vi "UHR-Fleezers Control (host) - 12.7c.vi"() -> ()   [LabVIEW 2012] (continued)
      tunnel: [w1052 _ _ _ w1081 _ w1113 _ _ w1145 _ w1159 _ _ w1229 w1232 w1242 w1245 w1315 _ w1336 w1361 w1381 w1402 w1422 w1447 w1477 _ w1484 w1579 w1584 w1622 _ w1657 w1661 w1665 w1676 w1680 _ w1688 _ _ _ _ _ _ _ _ _ _ _ _ _ _ _ _ _ w2066 _ _ _ _ w2107 _ _ _ _ _ _ _ _ _ _ _] -> w1011
      tunnel: w1010 -> [w1051 _ _ _ w1090 _ w1112 _ _ w1145 _ w1179 _ _ w1228 w1231 w1241 w1244 w1320 _ w1335 w1360 w1382 w1403 w1423 w1452 w1478 w1481 w1485 w1580 w1585 w1623 _ w1658 w1662 w1673 w1677 w1681 _ w1689 _ _ _ _ _ _ _ _ _ _ _ _ _ _ _ _ _ w2067 _ w2084 _ w2091 w2109 _ w2116 w2124 w2139 w2155 w2161 _ w2170 _ w2189 _]
      tunnel: [_ _ _ _ _ _ _ _ _ w1144 _ _ _ _ _ _ _ _ _ _ _ _ _ _ _ _ _ _ _ _ _ _ _ _ _ _ _ _ _ _ _ _ _ _ _ _ _ _ _ _ _ _ _ _ _ _ _ _ _ _ _ _ _ _ _ _ _ _ _ _ _ _ _ _] -> w1009
      tunnel: [_ _ _ _ _ _ _ "Round T1 X" _ _ _ _ _ _ _ _ _ _ _ _ _ _ _ _ _ _ _ _ _ _ _ _ _ _ _ _ _ _ _ _ _ _ _ _ _ _ _ _ _ _ _ _ _ _ _ _ _ _ _ _ _ _ _ _ _ _ _ _ _ _ _ _ _ _] -> _
      tunnel: [_ _ _ "Adjust Scale\nto Mean" _ _ _ _ _ _ _ _ _ _ _ _ _ _ _ _ _ _ _ _ _ _ _ _ "Test ttrig" _ _ _ _ _ _ _ _ _ _ _ _ _ _ _ _ _ _ "Flush Sample" "Flush Pump 3" "Flush Pump 1" "Clear Volume" _ _ _ _ _ _ _ _ _ _ _ _ _ _ _ _ _ _ _ _ _ _ _] -> _
      tunnel: [_ _ _ _ _ _ _ _ "Round T2 X" _ "Delayed Interlace Start" _ _ _ _ _ _ _ _ _ _ _ _ _ _ _ _ _ _ _ _ _ _ _ _ _ _ _ _ _ _ _ _ _ _ _ _ _ _ _ _ _ _ _ _ _ _ _ _ _ _ _ _ _ _ _ _ _ _ _ _ _ _ _] -> _
      tunnel: w1008 -> [_ _ _ _ _ _ _ _ _ _ _ _ _ _ _ _ _ _ _ _ _ _ _ _ _ _ _ _ _ _ _ _ _ _ _ _ _ _ _ _ _ _ _ w1847 w1854 w1861 w1866 w1875 _ _ w1981 _ _ _ _ _ _ _ _ _ _ _ _ _ _ _ _ _ _ _ _ _ _ _]
      tunnel: w1007 -> [_ _ _ _ _ _ _ _ _ _ _ _ _ _ _ _ _ _ _ _ _ _ _ _ _ _ _ _ _ _ _ _ _ _ _ _ _ _ _ _ _ w1764 _ _ _ _ _ _ w1919 _ _ w1987 _ w1996 _ w2010 _ _ _ _ _ _ _ _ _ _ _ _ _ _ _ _ _ _]
      tunnel: w1006 -> [_ _ _ _ _ _ _ _ _ _ _ _ _ _ _ _ _ _ _ _ _ _ _ _ _ _ _ _ _ _ _ _ _ _ _ _ _ _ _ _ _ _ _ _ _ _ _ _ _ _ _ _ _ _ _ _ _ _ _ _ _ _ _ _ _ _ _ _ _ _ _ _ _ _]
      tunnel: w1005 -> [_ _ _ _ _ _ _ _ _ _ _ _ _ _ _ _ _ _ _ _ _ _ _ _ _ _ _ _ _ _ _ _ _ _ _ _ _ _ _ _ w1701 _ _ _ _ _ _ _ _ w1949 _ _ w1992 _ w2003 _ w2035 _ _ _ _ _ _ _ _ _ _ _ _ _ _ _ _ _]
      tunnel: w1004 -> [_ _ _ _ _ _ _ _ _ _ _ _ _ _ _ _ _ _ _ _ _ _ _ _ _ _ _ _ _ _ _ _ _ _ _ _ _ _ _ _ _ _ _ _ _ _ _ _ _ _ _ _ _ _ _ _ _ _ _ _ _ _ _ _ _ _ _ _ _ _ _ _ _ _]
      event "AI Count (ticks)", "Sets to FIFO (Traps)", "Save ave N", "FPGA Ave.", "# Samples/channel", "N sets to save": Value Change {
        # "So that if 'Save ave N' is updated, the AOD scanning code updates too."
        n732 = event-data() -> ()  [unwired: 6 out]
        n733 = local read "AI Count (ticks)"() -> (w1035:u16)
        n734 = Unbundle By Name("Sets to FIFO (Traps)") -> ("Set 1"=w1018:bool, "Set 2"=w1017:bool, "Set 3"=w1016:bool)
        n735 = Boolean To (0,1)(Boolean="Sets to FIFO (Traps)") -> (0, 1=w1043:cluster{"Set 1":i16, "Set 2":i16, "Set 3":i16})
        n736 = xnode "Read/Write Control"("FPGA VI Reference In"=w1053, "error in"=w1051, "ai count"=w1035, "Set 1"=w1018, "Set 2"=w1017, "Set 3"=w1016, "N of AI1 Int Acq Sets"="N Acq Sets (Traps + Fl.)") -> ("error out"=w1052:errorcluster)  [unwired: 1 out]
        n737 = Cluster To Array(cluster=w1043) -> (array=w1042:i16[])
        n738 = To Unsigned Long Integer(number=w1042) -> (unsigned 32bit integer=w1024:u32[])
        n739 = local read "Scan steps (AOD)"() -> (w1044:u64)
        n740 = Multiply(x=w1035, y="N Acq Sets (Traps + Fl.)") -> (x*y=w1033:u16)
        n741 = Divide(x=40000000.0, y=w1035) -> (x/y=w1027:dbl)
        "AI rate (Hz)" <- w1027
        "Ave. Rate (Hz)" <- w1027
        n742 = Add Array Elements(numeric array=w1024) -> (sum=w1036:u32)
        "Trap Sets" <- w1036
        n743 = Reciprocal(x=w1027) -> (1/x=→"Ave. Period (s)":dbl)
        n744 = property on="Scan steps (AOD)" class="DigNum (strict)"("Val(Sgnl)"=w1044) -> ()  [unwired: 2 in, 2 out]
        n745 = Divide(x=w1027, y="N Acq Sets (Traps + Fl.)") -> (x/y=w1048:dbl)
        "Data Rate (Hz)" <- w1048
        n746 = Reciprocal(x=w1048) -> (1/x=→"Data Period (s)":dbl)
        n747 = local read "Save ave N"() -> (w1047:dbl)
        n748 = Divide(x=w1048, y=w1047) -> (x/y=w1046:dbl)
        "Save Data Rate (Hz)" <- w1046
        n749 = Reciprocal(x=w1046) -> (1/x=→"Save Data Period (s)":dbl)
        n750 = Multiply(x=w1033, y="# Samples/trap") -> (x*y=w1031:u32)
        "Counts/DMA" <- w1031
        n751 = property on="Trap Disp. Downsample" class="DigNum (strict)"("Maximum"="# Samples/trap") -> ()  [unwired: 2 in, 2 out]
        n752 = Multiply(x=w1036, y="# Samples/trap") -> (x*y=w1025:u32)
        "# Samples/channel" <- w1025
        n753 = Multiply(x=w1025, y=u32 8) -> (x*y=→"Trap AI Elements/DMA read":u32)
        n754 = local read "APD Int. Count"() -> (w1032:u32)
        n755 = Multiply(x=w1025, y=u32 3) -> (x*y=→"Trap Pos Elements/DMA read":u32)
        n756 = Divide(x=w1031, y=w1032) -> (x/y=w1022:dbl)
        "APD Samples/FIFO Acq." <- w1022
        n757 = Divide(x=w1031, y=40000000.0) -> (x/y=w1029:dbl)
        "DMA Update Period (s)" <- w1029
        n758 = local read "Number of APDs"() -> (w1015:u8)
        n759 = Multiply(x=w1015, y=w1022) -> (x*y=→"APD Elements/DMA read":dbl)
        n760 = property on="APD Disp. Downsample" class="DigNum (strict)"("Maximum"=w1022) -> ()  [unwired: 2 in, 2 out]
        n761 = local read "N sets to save"() -> (w1041:u32)
        n762 = Multiply(x=w1029, y=w1041) -> (x*y=→"Total Time (s)":dbl)
        "FPGA Averaging" <- FALSE ("FPGA Averaging")
      }
      event "Remove Offset": Value Change {
        n763 = event-data() -> ()  [unwired: 7 out]
        n764 = local write "Remove Offset"(FALSE ("Remove Offset")) -> ()
        n765 = local read "Bead Mean (nm)"() -> (w1055:dbl)
        n766 = local read "Offset (nm)"() -> (w1056:dbl)
        n767 = Add(x=w1055, y=w1056) -> (x+y=w1054:dbl)
        n768 = local write "Offset (nm)"(w1054) -> ()
        n769 = disable-structure shown="Disabled" {
          frame Disabled {
            n770 = local read "Bead Mean (nm)"() -> (w1061:dbl)
            n771 = Add(y=w1061) -> (x=w1060:dbl, x+y=w1059:dbl)
            n772 = Subtract(x=w1061, y=w1060) -> (x-y=w1058:dbl)
            n773 = property on="Bead Separation" class="WFChart (strict)"("YScale.Minimum"=w1058) -> ()  [unwired: 2 in, 2 out]
            n774 = property on="Bead Separation" class="WFChart (strict)"("YScale.Maximum"=w1059) -> ()  [unwired: 2 in, 2 out]
          }
          frame Enabled {
          }
        }
      }
      event "Detector Type": Value Change {
        n775 = event-data() -> ()  [unwired: 7 out]
        n776 = local read "AI labels"() -> (w1062:string[])
        n777 = property on="High Res. Display" class="Ring (strict)"("Strings []"=w1062) -> ()  [unwired: 2 in, 2 out]
        n778 = Build Array (concatenate)(w1062, "none") -> (w1063:string[])
        n779 = property on="FFT 1 Choice 1" class="Ring (strict)"("Strings []"=w1063) -> ()  [unwired: 2 in, 2 out]
        n780 = property on="FFT 1 Choice 2" class="Ring (strict)"("Strings []"=w1063) -> ()  [unwired: 2 in, 2 out]
        n781 = property on="FFT 2 Choice 1" class="Ring (strict)"("Strings []"=w1063) -> ()  [unwired: 2 in, 2 out]
        n782 = property on="FFT 2 Choice 2" class="Ring (strict)"("Strings []"=w1063) -> ()  [unwired: 2 in, 2 out]
        n783 = Bundle("APD 1", "APD 2") -> (w1066:cluster{string, string})  [unwired: 1 out]
        n784 = Cluster To Array(cluster=w1066) -> (array=w1064:string[])
        n785 = Build Array (concatenate)(w1064, w1063) -> (w1068:string[])
        n786 = Array Size(array=w1068) -> (size(s)=w1069:i32)
        n787 = property on="Signals to Plot" class="LstBox (strict)"("Item Names"=w1068) -> ()  [unwired: 2 in, 2 out]
        n788 = property on="Signals to Plot" class="LstBox (strict)"("Number of Rows"=w1069) -> ()  [unwired: 2 in, 2 out]
        n789 = property on="All Signals" class="WFChart (strict)"("LegNumRows"=w1069) -> ()  [unwired: 2 in, 2 out]
      }
      event "Adjust Scale\nto Mean": Value Change {
        n790 = event-data() -> ()  [unwired: 7 out]
        n791 = local read "APD 1 Rate (Hz)"() -> (w1078:dbl)
        n792 = Multiply(x=1000.0, y="Above (kHz)") -> (x*y=w1076:dbl)
        n793 = Multiply(x=1000.0, y="Below (kHz)") -> (x*y=w1074:dbl)
        n794 = Add(x=w1076, y=w1078) -> (x+y=w1071:dbl)
        n795 = Subtract(x=w1078, y=w1074) -> (x-y=w1072:dbl)
        n796 = property on="APD Chart" class="WFChart (strict)"("YScale.Minimum"=w1072) -> ()  [unwired: 2 in, 2 out]
        n797 = property on="APD Chart" class="WFChart (strict)"("YScale.Maximum"=w1071) -> ()  [unwired: 2 in, 2 out]
      }
      event "Phase adj. (AI1)", "+ phase (AI1)", "- phase (AI1)": Value Change {
        n798 = event-data() -> ()  [unwired: 7 out]
        n799 = Negate(x="Phase adj. (AI1)") -> (-x=w1088:i16)
        n800 = Select(t=w1088, s="- phase (AI1)", f="Phase adj. (AI1)") -> (s? t:f=w1087:i16)
        n801 = xnode "Read/Write Control"("FPGA VI Reference In"=w1091, "error in"=w1090, "Phase count adjustment"=w1087) -> ("FPGA VI Reference Out"=w1086:T20, "error out"=w1085:errorcluster)  [unwired: 1 in]
        n802 = Or(x="- phase (AI1)", y="+ phase (AI1)") -> (x .or. y?=w1082:bool)
        n803 = xnode "Read/Write Control"("FPGA VI Reference In"=w1086, "error in"=w1085, "+ phase"=w1082) -> ("error out"=w1081:errorcluster)  [unwired: 1 in, 1 out]
      }
      event "Signals to Plot": Double Click {
        w1094 = u32 9868950 ("Color Box")
        n804 = event-data() -> ("Row"=w1096:i32)  [unwired: 9 out]
        n805 = property on="All Signals" class="WFChart (strict)"("Active Plot"=w1096) -> (error out=w1107:errorcluster)  [unwired: 2 in, 1 out]
        n806 = property on="All Signals" class="WFChart (strict)" props=["Plot", "Visible?", "Plot", "Plot Color"](error in=w1107) -> (error out=w1106:errorcluster, "Plot.Visible?"=w1105:bool)  [unwired: 1 in, 2 out]
        n807 = Select(t=FALSE ("Plot.Visible"), s=w1105, f=TRUE ("Plot.Visible")) -> (s? t:f=w1100:bool)
        n808 = property on="All Signals" class="WFChart (strict)"(error in=w1106, "Plot.Visible?"=w1100) -> (error out=w1102:errorcluster)  [unwired: 1 in, 1 out]
        n809 = property on="All Signals" class="WFChart (strict)"(error in=w1102) -> (error out=w1097:errorcluster, "Plot.Plot Color"=w1101:u32)  [unwired: 1 in, 1 out]
        n810 = property on="Signals to Plot" class="LstBox (strict)"(error in=w1097, "Active Row"=w1096) -> (error out=w1095:errorcluster)  [unwired: 1 in, 1 out]
        n811 = Select(t=w1101, s=w1100, f=u32 0) -> (s? t:f=w1098:u32)
        n812 = property on="Signals to Plot" class="LstBox (strict)"(error in=w1095, "CellFontColor"=w1098, "SelColor"=w1094, "CellBG"=w1094, "CellFontSize"=u32 20 ("Active Row:Cell Font:Size"), "CellFontBold"=TRUE ("Active Row:Cell Font:Bold")) -> ()  [unwired: 1 in, 2 out]
      }
      event "BD 1 Frequency 1 (MHz)", "BD 1 Frequency 2 (MHz)", "BD 1 Frequency 3 (MHz)", "BD 2 Frequency 1 (MHz)", "BD 2 Frequency 2 (MHz)", "BD 2 Frequency 3 (MHz)", "Trap Delta (MHz)", "Update all trap values": Value Change {
        # "This is so you can set trap frequencies\nvia local variables and then update\nall at once"
        n813 = event-data() -> ("CtlRef"=w1111:refnum<vi>)  [unwired: 6 out]
        n814 = control-ref of="Trap Delta (MHz)"() -> (w1110:refnum<vi>)
        n815 = Equal?(x=w1110, y=w1111) -> (x = y?=w1109:bool)
        n816 = local write "Update all trap values"(FALSE ("Update all trap values")) -> ()
        n817 = case shown="False" "Oscillate Set 1" {
          tunnel: w1114 -> [w1134 _]
          tunnel: [w1133 w1137] -> w1113
          tunnel: w1112 -> [w1132 w1137]
          tunnel: w1109 -> [w1117 _]
          frame False {
            n818 = local read "BD 1 Frequency 2 (MHz)"() -> (w1121:dbl)
            n819 = local read "BD 1 Frequency 1 (MHz)"() -> (w1119:dbl)
            n820 = Subtract(x=w1121, y="Trap Delta (MHz)") -> (x-y=w1118:dbl)
            n821 = Select(t=w1118, s=w1117, f=w1119) -> (s? t:f=w1116:dbl)
            n822 = local read "Y RF Frequency Limits (MHz)"() -> (w1122:T16)
            n823 = local read "X RF Frequency Limits (MHz)"() -> (w1123:T16)
            n824 = local write "BD 1 Frequency 1 (MHz)"(w1116) -> ()
            n825 = local read "BD 1 Frequency 3 (MHz)"() -> (w1135:dbl)
            n826 = local read "BD 2 Frequency 1 (MHz)"() -> (w1126:dbl)
            n827 = local read "BD 2 Frequency 2 (MHz)"() -> (w1125:dbl)
            n828 = local read "BD 2 Frequency 3 (MHz)"() -> (w1136:dbl)
            n829 = call "set RF board frequency - interlace.vi"("Board 2 Frequency Limits"=w1122, "Board 1 Frequency Limits"=w1123, "error in"=w1132, "FPGA VI Reference In"=w1134, "Board 2 Frequency 3 (MHz)"=w1136, "Board 1 Frequency 3 (MHz)"=w1135, "Board 2 Frequency 2 (MHz)"=w1125, "Board 2 Frequency 1 (MHz)"=w1126, "Board 1 Frequency 2 (MHz)"=w1121, "Board 1 Frequency 1  (MHz)"=w1116) -> ("error out"=w1133:errorcluster)  [unwired: 1 out]
            n830 = Subtract(x=w1126, y=w1125) -> (x-y=w1130:dbl)
            n831 = Subtract(x=w1116, y=w1121) -> (x-y=w1131:dbl)
            n832 = Square(x=w1130) -> (x^2=w1128:dbl)
            n833 = Square(x=w1131) -> (x^2=w1129:dbl)
            n834 = Add(x=w1129, y=w1128) -> (x+y=w1127:dbl)
            n835 = Square Root(x=w1127) -> (sqrt(x)=w1124:dbl)
            n836 = property on="Initial delta (MHz)" class="DigNum (strict)"("Val(Sgnl)"=w1124) -> ()  [unwired: 2 in, 2 out]
            n837 = local write "Trap Delta (MHz)"(w1124) -> ()
          }
          frame True {
          }
        }
      }
      event "Round T1 X": Value Change {
        n838 = event-data() -> ()  [unwired: 7 out]
        n839 = local read "BD 1 Frequency 1 (MHz)"() -> (w1140:dbl)
        n840 = Round To Nearest(number=w1140) -> (nearest integer value=w1139:dbl)
        n841 = property on="BD 1 Frequency 1 (MHz)" class="DigNum (strict)"("Val(Sgnl)"=w1139) -> ()  [unwired: 2 in, 2 out]
      }
      event "Round T2 X": Value Change {
        n842 = event-data() -> ()  [unwired: 7 out]
        n843 = local read "BD 1 Frequency 2 (MHz)"() -> (w1142:dbl)
        n844 = Round To Nearest(number=w1142) -> (nearest integer value=w1141:dbl)
        n845 = property on="BD 1 Frequency 2 (MHz)" class="DigNum (strict)"("Val(Sgnl)"=w1141) -> ()  [unwired: 2 in, 2 out]
      }
      event "Stop All": Value Change {
        n846 = event-data() -> ()  [unwired: 7 out]
        n847 = local read "Stop All"() -> (w1144:bool)
      }
      event "Delayed Interlace Start": Value Change {
        n848 = event-data() -> ()  [unwired: 7 out]
        n849 = flat-sequence {
          frame #0 {
            n850 = Multiply(x="Delay to Interlace (s)", y=1000.0) -> (x*y=w1147:dbl)
            n851 = Wait (ms)(milliseconds to wait=w1147) -> ()  [unwired: 1 out]
          }
          frame #1 {
            n852 = property on="Laser interlacing mode" class="RadioBtnsControl (strict)"("Val(Sgnl)"=enum32{"Laser ON", "Laser OFF", "Interlace"}."Interlace" ("Value (Signaling)")) -> ()  [unwired: 2 in, 2 out]
          }
        }
      }
      event "BD 1 Amplitude 1 (%)", "BD 1 Amplitude 2 (%)", "BD 1 Amplitude 3 (%)", "BD 2 Amplitude 1 (%)", "BD 2 Amplitude 2 (%)", "BD 2 Amplitude 3 (%)", "Trap 1 ON", "Trap 2 ON", "Trap 3 ON", "Feedback On/Off", "All FB On/Off": Value Change {
        w1171 = i16 1 ("f")
        n853 = event-data() -> ()  [unwired: 7 out]
        n854 = local write "Trap 1 (ON/OFF)"("Trap 1 ON") -> ()
        n855 = local write "Trap 2 (ON/OFF)"("Trap 2 ON") -> ()
        n856 = Boolean To (0,1)(Boolean="Trap 3 ON") -> (0, 1=w1172:i16)
        n857 = Boolean To (0,1)(Boolean="Trap 1 ON") -> (0, 1=w1173:i16)
        n858 = Boolean To (0,1)(Boolean="Trap 2 ON") -> (0, 1=w1174:i16)
        n859 = Select(t=w1174, s="Trap ON/OFF X or Y Amp?", f=w1171) -> (s? t:f=w1169:i16)
        n860 = Select(t=w1173, s="Trap ON/OFF X or Y Amp?", f=w1171) -> (s? t:f=w1170:i16)
        n861 = Select(t=w1172, s="Trap ON/OFF X or Y Amp?", f=w1171) -> (s? t:f=w1168:i16)
        n862 = Select(t=w1171, s="Trap ON/OFF X or Y Amp?", f=w1174) -> (s? t:f=w1166:i16)
        n863 = Select(t=w1171, s="Trap ON/OFF X or Y Amp?", f=w1173) -> (s? t:f=w1167:i16)
        n864 = Select(t=w1171, s="Trap ON/OFF X or Y Amp?", f=w1172) -> (s? t:f=w1165:i16)
        n865 = And(x="All FB On/Off", y="Feedback On/Off") -> (x .and. y?=w1163:cluster{"Set 1":bool, "Set 2":bool})
        n866 = local read "BD 1 Amplitude 1 (%)"() -> (w1183:dbl)
        n867 = local read "BD 1 Amplitude 2 (%)"() -> (w1182:dbl)
        n868 = local read "BD 1 Amplitude 3 (%)"() -> (w1181:dbl)
        n869 = Unbundle By Name(w1163) -> ("Set 1"=w1158:bool, "Set 2"=w1155:bool)
        n870 = local read "Y RF Amplitude Limits (%)"() -> (w1151:T16)
        n871 = local read "X RF Amplitude Limits (%)"() -> (w1152:T16)
        n872 = local read "BD 2 Amplitude 1 (%)"() -> (w1184:dbl)
        n873 = local read "BD 2 Amplitude 2 (%)"() -> (w1185:dbl)
        n874 = local read "BD 2 Amplitude 3 (%)"() -> (w1186:dbl)
        n875 = And(x="Trap 2 ON", y=w1155) -> (x .and. y?=w1153:bool)
        n876 = And(x="Trap 1 ON", y=w1158) -> (x .and. y?=w1156:bool)
        n877 = Multiply(x=w1170, y=w1183) -> (x*y=w1178:dbl)
        n878 = Multiply(x=w1182, y=w1169) -> (x*y=w1176:dbl)
        n879 = Multiply(x=w1181, y=w1168) -> (x*y=w1177:dbl)
        n880 = Multiply(x=w1184, y=w1167) -> (x*y=w1187:dbl)
        n881 = Multiply(x=w1185, y=w1166) -> (x*y=w1188:dbl)
        n882 = Multiply(x=w1186, y=w1165) -> (x*y=w1189:dbl)
        n883 = call "set RF board amplitude - interlace.vi"("Board 2 Amplitude Limits"=w1151, "Board 1 Amplitude Limits"=w1152, "error in"=w1179, "FPGA VI Reference In"=w1180, "Board 2 Amplitude 3 (%)"=w1189, "Board 1 Amplitude 3 (%)"=w1177, "Board 2 Amplitude 2 (%)"=w1188, "Board 2 Amplitude 1 (%)"=w1187, "Board 1 Amplitude 2 (%)"=w1176, "Board 1 Amplitude 1 (%)"=w1178) -> ("error out"=w1160:errorcluster, "FPGA VI Reference Out"=w1161:T20)
        n884 = xnode "Read/Write Control"("FPGA VI Reference In"=w1161, "error in"=w1160, "FB On/Off Set 1"=w1156, "FB On/Off Set 2"=w1153) -> ("error out"=w1159:errorcluster)  [unwired: 1 out]
      }
      event "Load parameters": Value Change {
        n885 = event-data() -> ()  [unwired: 7 out]
        n886 = property on="Saved AOD Raster Scan Parameter Sets" class="Arr (strict)"() -> ("Index Values"=w1200:u32[])  [unwired: 2 in, 2 out]
        n887 = Index Array(array=w1200, index=0) -> (element=w1197:u32)
        n888 = local write "Load parameters"(FALSE ("Load parameters")) -> ()
        n889 = Index Array(array="Saved AOD Raster Scan Parameter Sets", index=w1197) -> (element=w1196:T28)
        n890 = Unbundle By Name(w1196) -> ("Scan Range AOD (nm) 2"=w1195:dbl, "Step Size AOD (nm) 2"=w1194:dbl, "Scan Speed AOD (nm/s) 2"=w1193:dbl, "Number of scans (AOD) 2"=w1192:u16)
        n891 = flat-sequence {
          tunnel: w1195 -> [w1203]
          tunnel: w1194 -> [w1202]
          tunnel: w1193 -> [w1201]
          tunnel: w1192 -> [w1204]
          frame #0 {
            n892 = local write "Scan Speed (nm/s)"(w1201) -> ()
            n893 = local write "Scan Range (nm)"(w1203) -> ()
            n894 = local write "Step Size (nm)"(w1202) -> ()
          }
          frame #1 {
            n895 = property on="Number of F/B Scans (AOD)" class="DigNum (strict)"("Val(Sgnl)"=w1204) -> ()  [unwired: 2 in, 2 out]
          }
        }
      }
      event "Trap 1 (ON/OFF)", "Trap 2 (ON/OFF)": Value Change {
        n896 = event-data() -> ()  [unwired: 7 out]
        n897 = property on="Trap 2 ON" class="Bool (strict)"("Val(Sgnl)"="Trap 2 (ON/OFF)") -> ()  [unwired: 2 in, 2 out]
        n898 = property on="Trap 1 ON" class="Bool (strict)"("Val(Sgnl)"="Trap 1 (ON/OFF)") -> ()  [unwired: 2 in, 2 out]
      }
      event "DIO count 1 (ticks)", "DIO count 2 (ticks)", "DIO count 3 (ticks)", "Interlace", "Number Interlace Sets", "Not-Interlacing Set", "BD 1 Delay (ticks)", "BD 2 Delay (Ticks)", "Next trap write delay (ticks)", "XY phase ext loop method", "Amp switch delay 2", "BD 2 Delay (Ticks) 2", "BD 1 Delay (ticks) 2": Value Change {
        n899 = event-data() -> ()  [unwired: 7 out]
        n900 = local read "DIO count 3 (ticks)"() -> (w1224:u16)
        n901 = local read "DIO count 1 (ticks)"() -> (w1226:u16)
        n902 = local read "DIO count 2 (ticks)"() -> (w1225:u16)
        n903 = To Unsigned Byte Integer(number="Not-Interlacing Set") -> (unsigned 8bit integer=w1215:u8)
        n904 = Add(x=w1215, y=u8 1) -> (x+y=w1219:u8)
        n905 = xnode "Read/Write Control"("FPGA VI Reference In"=w1230, "error in"=w1228, "DIO count 1 (ticks)"=w1226, "DIO count 2 (ticks)"=w1225, "DIO count 3 (ticks)"=w1224, "Interlace ON/OFF"="Interlace", "Number Interlace Cycles"="Number Interlace Sets", "Interlace Off Parameters"=w1219, "BD 1 Delay (ticks)"="BD 1 Delay (ticks)", "BD 2 Delay (Ticks)"="BD 2 Delay (Ticks)", "Next trap write delay (ticks)"="Next trap write delay (ticks)", "XY phase ext loop method"="XY phase ext loop method", "Amp switch delay 2"="Amp switch delay 2", "BD 2 Delay (Ticks) 2"="BD 2 Delay (Ticks) 2", "BD 1 Delay (ticks) 2"="BD 1 Delay (ticks) 2") -> ("error out"=w1229:errorcluster)  [unwired: 1 out]
        n906 = Build Array(w1226, w1225, w1224) -> (w1217:u16[])
        n907 = Split 1D Array(array=w1217, index="Number Interlace Sets") -> (first subarray=w1227:u16[])  [unwired: 1 out]
        n908 = Index Array(array=w1217, index=w1215) -> (element=w1216:u16)
        n909 = Add Array Elements(numeric array=w1227) -> (sum=w1221:u16)
        n910 = Select(t=w1221, s="Interlace", f=w1216) -> (s? t:f=→"Total Counts (ticks)":u16)
      }
      event "Reset Feedback": Value Change {
        n911 = event-data() -> ()  [unwired: 7 out]
        n912 = Unbundle By Name("Reset Feedback") -> ("Set 1"=w1234:bool, "Set 2"=w1233:bool)
        n913 = xnode "Read/Write Control"("FPGA VI Reference In"=w1236, "error in"=w1231, "FB Reset Set 1"=w1234, "FB Reset Set 2"=w1233) -> ("error out"=w1232:errorcluster)  [unwired: 1 out]
      }
      event "Trap Intensity PID Gains": Value Change {
        n914 = event-data() -> ()  [unwired: 7 out]
        n915 = Unbundle By Name("Trap Intensity PID Gains") -> ("proportional gain (Kc)"=w1239:i16, "integral gain (Kc*Ts/Ti)"=w1238:i16, "derivative gain (Kc*Td/Ts)"=w1237:i16)
        n916 = xnode "Read/Write Control"("FPGA VI Reference In"=w1243, "error in"=w1241, "P1"=w1239, "I1"=w1238, "D1"=w1237) -> ("error out"=w1242:errorcluster)  [unwired: 1 out]
      }
      event "AI2 to Setpoint", "Setpoints (V)": Value Change {
        n917 = event-data() -> ()  [unwired: 7 out]
        n918 = xnode "Read/Write Control"("FPGA VI Reference In"=w1248, "error in"=w1244) -> ("FPGA VI Reference Out"=w1247:T20, "error out"=w1246:errorcluster, "AI2 Y Sum Set 1"=w1255:i16, "AI2 Y Sum Set 2"=w1254:i16)
        n919 = Cluster To Array(cluster="AI2 to Setpoint") -> (array=w1258:bool[])
        n920 = local read "AI2 (V)"() -> (w1256:cluster{"Set 1":dbl, "Set 2":dbl})
        n921 = Or Array Elements(Boolean array=w1258) -> (logical OR=w1259:bool)
        n922 = Bundle By Name(cluster=w1256, "Set 1"=w1255, "Set 2"=w1254) -> (w1253:cluster{"Set 1":dbl, "Set 2":dbl})
        n923 = Divide(x=w1253, y=3276.7) -> (x/y=w1252:cluster{"Set 1":dbl, "Set 2":dbl})
        "AI2 (V)" <- w1252
        n924 = case shown="True" w1259 {
          tunnel: [w1262 w1279] -> w1251
          tunnel: "AI2 to Setpoint" -> [_ w1275]
          tunnel: "Setpoints (V)" -> [w1263 w1278]
          tunnel: w1252 -> [_ w1272]
          frame False {
            n925 = Multiply(x=3276.7, y=w1263) -> (x*y=w1264:cluster{"Set 1":dbl, "Set 2":dbl})
            n926 = To Word Integer(number=w1264) -> (16bit integer=w1262:cluster{"Set 1":i16, "Set 2":i16})
          }
          frame True {
            n927 = Unbundle By Name(w1272) -> ("Set 1"=w1271:dbl, "Set 2"=w1270:dbl)
            n928 = Unbundle By Name(w1278) -> ("Set 1"=w1277:dbl, "Set 2"=w1276:dbl)
            n929 = Unbundle By Name(w1275) -> ("Set 1"=w1274:bool, "Set 2"=w1273:bool)
            n930 = Select(t=w1271, s=w1274, f=w1277) -> (s? t:f=w1269:dbl)
            n931 = Select(t=w1270, s=w1273, f=w1276) -> (s? t:f=w1268:dbl)
            n932 = Bundle By Name(cluster=w1278, "Set 1"=w1269, "Set 2"=w1268) -> (w1266:cluster{"Set 1":dbl, "Set 2":dbl})
            n933 = local write "Setpoints (V)"(w1266) -> ()
            n934 = Multiply(x=3276.7, y=w1266) -> (x*y=w1267:cluster{"Set 1":dbl, "Set 2":dbl})
            n935 = To Word Integer(number=w1267) -> (16bit integer=w1279:cluster{"Set 1":i16, "Set 2":i16})
          }
        }
        n936 = Unbundle By Name(w1251) -> ("Set 1"=w1250:i16, "Set 2"=w1249:i16)
        n937 = xnode "Read/Write Control"("FPGA VI Reference In"=w1247, "error in"=w1246, "FB Setpoint Set 1"=w1250, "FB Setpoint Set 2"=w1249) -> ("error out"=w1245:errorcluster)  [unwired: 1 out]
      }
      event "+ phase (GI)", "- phase (GI)", "+ phase (GI) 2", "- phase (GI) 2", "+ phase (RI)", "- phase (RI)", "+ phase (Green FB)", "- phase (Green FB)": Value Change {
        n938 = event-data() -> ()  [unwired: 7 out]
        n939 = Or(x="+ phase (GI)", y="- phase (GI)") -> (x .or. y?=w1314:bool)
        n940 = Negate(x="Phase adj. (GI)") -> (-x=w1319:i16)
        n941 = Select(t=w1319, s="+ phase (GI)", f="Phase adj. (GI)") -> (s? t:f=w1318:i16)
        n942 = Or(x="+ phase (GI) 2", y="- phase (GI) 2") -> (x .or. y?=w1305:bool)
        n943 = Negate(x="Phase adj. (GI) 2") -> (-x=w1310:i16)
        n944 = Select(t=w1310, s="+ phase (GI) 2", f="Phase adj. (GI) 2") -> (s? t:f=w1306:i16)
        n945 = Negate(x="Phase adj. (RI)") -> (-x=w1304:i16)
        n946 = Or(x="+ phase (RI)", y="- phase (RI)") -> (x .or. y?=w1300:bool)
        n947 = Select(t=w1304, s="+ phase (RI)", f="Phase adj. (RI)") -> (s? t:f=w1299:i16)
        n948 = Or(x="+ phase (Green FB)", y="- phase (Green FB)") -> (x .or. y?=w1293:bool)
        n949 = Negate(x="Phase adj. (Green FB)") -> (-x=w1298:i16)
        n950 = Select(t=w1298, s="+ phase (Green FB)", f="Phase adj. (Green FB)") -> (s? t:f=w1294:i16)
        n951 = Negate(x="Phase adj. (BI AO)") -> (-x=w1292:i16)
        n952 = Or(x="+ phase (BI AO)", y="- phase (BI AO)") -> (x .or. y?=w1282:bool)
        n953 = Select(t=w1292, s="+ phase (BI AO)", f="Phase adj. (BI AO)") -> (s? t:f=w1284:i16)
        n954 = Negate(x="Phase adj. (BI DO)") -> (-x=w1288:i16)
        n955 = Or(x="+ phase (BI DO)", y="- phase (BI DO)") -> (x .or. y?=w1281:bool)
        n956 = Select(t=w1288, s="+ phase (BI DO)", f="Phase adj. (BI DO)") -> (s? t:f=w1283:i16)
        n957 = xnode "Read/Write Control"("FPGA VI Reference In"=w1321, "error in"=w1320, "Phase count adjustment (GI)"=w1318, "Phase count adjustment (GI) 2"=w1306, "Phase count adjustment (RI)"=w1299, "Phase count adjustment (Green FB)"=w1294, "Phase count adjustment (BI AO)"=w1284, "Phase count adjustment (BI D)"=w1283) -> ("FPGA VI Reference Out"=w1316:T20, "error out"=w1317:errorcluster)
        n958 = xnode "Read/Write Control"("FPGA VI Reference In"=w1316, "error in"=w1317, "+ phase (GI)"=w1314, "+ phase (GI) 2"=w1305, "+ phase (RI)"=w1300, "+ phase (Green FB)"=w1293, "+ phase (BI AO)"=w1282, "+ phase (BI D)"=w1281) -> ("error out"=w1315:errorcluster)  [unwired: 1 out]
      }
      event "Green Laser ON/OFF", "Red Laser ON/OFF", "Blue Laser ON/OFF": Value Change {
        # "This loop shouldn't be initialized.  The main 'laser ON' settings should dominate and set the others."
        n959 = event-data() -> ()  [unwired: 7 out]
        n960 = property on="Red Laser ON" class="Bool (strict)"("Val(Sgnl)"="Red Laser ON/OFF") -> ()  [unwired: 2 in, 2 out]
        n961 = property on="Blue Laser ON" class="Bool (strict)"("Val(Sgnl)"="Blue Laser ON/OFF") -> ()  [unwired: 2 in, 2 out]
        n962 = property on="Green Laser ON" class="Bool (strict)"("Val(Sgnl)"="Green Laser ON/OFF") -> ()  [unwired: 2 in, 2 out]
      }
      event "Laser interlacing mode", "Green Laser ON", "Red Laser ON", "Blue Laser ON": Value Change {
        n963 = event-data() -> ()  [unwired: 7 out]
        n964 = local write "Green Laser ON/OFF"("Green Laser ON") -> ()
        n965 = local write "Blue Laser ON/OFF"("Blue Laser ON") -> ()
        n966 = local write "Red Laser ON/OFF"("Red Laser ON") -> ()
        n967 = case shown="True" "Green Laser ON" {
          tunnel: "Laser interlacing mode" -> [_ w1358]
          tunnel: [enum32{"Laser ON", "Laser OFF", "Interlace"}."Laser OFF" ("Green laser mode") w1358] -> w1334
          tunnel: [FALSE w1354] -> w1333
          frame False {
          }
          frame True {
            n968 = local read "Green FB On/Off"() -> (w1355:bool)
            n969 = Equal?(x=w1358, y=enum32{"Laser ON", "Laser OFF", "Interlace"}."Interlace") -> (x = y?=w1356:bool)
            n970 = And(x=w1356, y=w1355) -> (x .and. y?=w1354:bool)
          }
        }
        n971 = case shown="True" "Red Laser ON" {
          tunnel: "Laser interlacing mode" -> [_ w1351]
          tunnel: [enum32{"Laser ON", "Laser OFF", "Interlace"}."Laser OFF" ("Green laser mode") w1351] -> w1330
          tunnel: [FALSE w1347] -> w1329
          frame False {
          }
          frame True {
            n972 = local read "Red FB On/Off"() -> (w1348:bool)
            n973 = Equal?(x=w1351, y=enum32{"Laser ON", "Laser OFF", "Interlace"}."Interlace") -> (x = y?=w1349:bool)
            n974 = And(x=w1349, y=w1348) -> (x .and. y?=w1347:bool)
          }
        }
        n975 = case shown="True" "Blue Laser ON" {
          tunnel: "Laser interlacing mode" -> [_ w1342]
          tunnel: [enum32{"Laser ON", "Laser OFF", "Interlace"}."Laser OFF" ("Green laser mode") w1342] -> w1326
          tunnel: [FALSE w1340] -> w1325
          frame False {
          }
          frame True {
            n976 = local read "Blue FB On/Off"() -> (w1341:bool)
            n977 = Equal?(x=w1342, y=enum32{"Laser ON", "Laser OFF", "Interlace"}."Interlace") -> (x = y?=w1343:bool)
            n978 = And(x=w1343, y=w1341) -> (x .and. y?=w1340:bool)
          }
        }
        n979 = xnode "Read/Write Control"("FPGA VI Reference In"=w1337, "error in"=w1335, "Operating Mode"=w1334, "Operating Mode 2"=w1334, "Green FB On/Off"=w1333, "Red Laser Operating Mode"=w1330, "RI Operating Mode 2"=w1330, "Red FB On/Off"=w1329, "BI Operating Mode (AO)"=w1326, "Blue Laser Operating Mode (D)"=w1326, "Blue FB On/Off"=w1325) -> ("error out"=w1336:errorcluster)  [unwired: 1 out]
      }
      event "Invert laser interlacing": Value Change {
        n980 = event-data() -> ()  [unwired: 7 out]
        n981 = xnode "Read/Write Control"("FPGA VI Reference In"=w1362, "error in"=w1360, "Invert GI"="Invert laser interlacing", "Invert GI 2"="Invert laser interlacing", "Invert RI"="Invert laser interlacing", "Invert RI 2"="Invert laser interlacing", "Invert BI (AO)"="Invert laser interlacing", "Invert BI (D)"="Invert laser interlacing") -> ("error out"=w1361:errorcluster)  [unwired: 1 out]
      }
      event "Green FB Setpoint (mV)", "Green FB Gains", "Green FB On/Off", "Green Intensity % (FB OFF)", "Green int current ON count adj": Value Change {
        n982 = event-data() -> ()  [unwired: 7 out]
        n983 = local read "Green FB Setpoint (mV)"() -> (w1373:dbl)
        n984 = Multiply(x=w1373, y=3.2767) -> (x*y=w1372:dbl)
        n985 = local read "Green Intensity % (FB OFF)"() -> (w1376:dbl)
        n986 = Multiply(x=w1376, y=655.35) -> (x*y=w1377:dbl)
        n987 = To Unsigned Word Integer(number=w1377) -> (unsigned 16bit integer=w1375:u16)
        n988 = local read "Green int current ON count adj"() -> (w1379:u32)
        n989 = local read "Laser interlacing mode"() -> (w1369:enum32{"Laser ON", "Laser OFF", "Interlace"})
        n990 = local read "Green FB Gains"() -> (w1366:T9)
        n991 = local read "Green Laser ON"() -> (w1370:bool)
        n992 = local read "Green FB On/Off"() -> (w1380:bool)
        n993 = Equal?(x=w1369, y=enum32{"Laser ON", "Laser OFF", "Interlace"}."Interlace") -> (x = y?=w1367:bool)
        n994 = Unbundle By Name(w1366) -> ("proportional gain (Kc)"=w1365:i16, "integral gain (Kc*Ts/Ti)"=w1364:i16, "derivative gain (Kc*Td/Ts)"=w1363:i16)
        n995 = Compound Arithmetic op=AND(w1367, w1380, w1370) -> (w1371:bool)
        n996 = xnode "Read/Write Control"("FPGA VI Reference In"=w1383, "error in"=w1382, "Green FB Setpoint"=w1372, "Green FB On/Off"=w1371, "Current Out"=w1375, "Green int current ON count adj"=w1379, "P3"=w1365, "I3"=w1364, "D3"=w1363) -> ("error out"=w1381:errorcluster)  [unwired: 1 out]
      }
      event "Blue FB Setpoint (mV)", "Blue FB Gains", "Blue FB On/Off", "Blue Intensity % (FB OFF)", "Blue int AO ON count adjust": Value Change {
        # "16 bit analog out"
        n997 = event-data() -> ()  [unwired: 7 out]
        n998 = Multiply(x="Blue FB Setpoint (mV)", y=3.2767) -> (x*y=w1397:dbl)
        n999 = Multiply(x="Blue Intensity % (FB OFF)", y=655.35) -> (x*y=w1400:dbl)
        n1000 = To Unsigned Word Integer(number=w1400) -> (unsigned 16bit integer=w1399:u16)
        n1001 = local read "Laser interlacing mode"() -> (w1395:enum32{"Laser ON", "Laser OFF", "Interlace"})
        n1002 = Unbundle By Name("Blue FB Gains") -> ("proportional gain (Kc)"=w1392:i16, "integral gain (Kc*Ts/Ti)"=w1391:i16, "derivative gain (Kc*Td/Ts)"=w1390:i16)
        n1003 = local read "Blue Laser ON"() -> (w1384:bool)
        n1004 = Equal?(x=w1395, y=enum32{"Laser ON", "Laser OFF", "Interlace"}."Interlace") -> (x = y?=w1393:bool)
        n1005 = Compound Arithmetic op=AND(w1393, "Blue FB On/Off", w1384) -> (w1396:bool)
        n1006 = xnode "Read/Write Control"("FPGA VI Reference In"=w1404, "error in"=w1403, "Blue FB Setpoint"=w1397, "Blue FB On/Off"=w1396, "BI Current Out"=w1399, "Blue current ON count adj (AO)"="Blue int AO ON count adjust", "P5"=w1392, "I5"=w1391, "D5"=w1390) -> ("error out"=w1402:errorcluster)  [unwired: 1 out]
      }
      event "Red FB Setpoint (mV)", "Red FB Gains", "Red FB On/Off", "Red Intensity % (FB OFF)": Value Change {
        n1007 = event-data() -> ()  [unwired: 7 out]
        n1008 = local read "Red FB Setpoint (mV)"() -> (w1416:dbl)
        n1009 = Multiply(x=w1416, y=3.2767) -> (x*y=w1415:dbl)
        n1010 = local read "Red Intensity % (FB OFF)"() -> (w1405:dbl)
        n1011 = Multiply(x=w1405, y=655.35) -> (x*y=w1419:dbl)
        n1012 = To Unsigned Word Integer(number=w1419) -> (unsigned 16bit integer=w1418:u16)
        n1013 = local read "Laser interlacing mode"() -> (w1412:enum32{"Laser ON", "Laser OFF", "Interlace"})
        n1014 = local read "Red FB Gains"() -> (w1409:T9)
        n1015 = local read "Red Laser ON"() -> (w1413:bool)
        n1016 = local read "Red FB On/Off"() -> (w1421:bool)
        n1017 = Equal?(x=w1412, y=enum32{"Laser ON", "Laser OFF", "Interlace"}."Interlace") -> (x = y?=w1410:bool)
        n1018 = Unbundle By Name(w1409) -> ("proportional gain (Kc)"=w1408:i16, "integral gain (Kc*Ts/Ti)"=w1407:i16, "derivative gain (Kc*Td/Ts)"=w1406:i16)
        n1019 = Compound Arithmetic op=AND(w1410, w1421, w1413) -> (w1414:bool)
        n1020 = xnode "Read/Write Control"("FPGA VI Reference In"=w1424, "error in"=w1423, "Red FB Setpoint"=w1415, "Red FB On/Off"=w1414, "RI Current Out"=w1418, "P4"=w1408, "I4"=w1407, "D4"=w1406) -> ("error out"=w1422:errorcluster)  [unwired: 1 out]
      }
      event "+ phase (APD 1 Gate)", "- phase (APD 1 Gate)", "+ phase (APD 2 Gate)", "- phase (APD 2 Gate)", "+ phase (APD 3 Gate)", "- phase (APD 3 Gate)", "+ phase (APD Acq)", "- phase (APD Acq)": Value Change {
        n1021 = event-data() -> ()  [unwired: 7 out]
        n1022 = local read "Phase Adj. (APD 1 Gate)"() -> (w1444:i16)
        n1023 = Or(x="- phase (APD 1 Gate)", y="+ phase (APD 1 Gate)") -> (x .or. y?=w1446:bool)
        n1024 = Negate(x=w1444) -> (-x=w1451:i16)
        n1025 = Select(t=w1451, s="+ phase (APD 1 Gate)", f=w1444) -> (s? t:f=w1450:i16)
        n1026 = local read "Phase Adj. (APD 2 Gate)"() -> (w1441:i16)
        n1027 = Or(x="- phase (APD 2 Gate)", y="+ phase (APD 2 Gate)") -> (x .or. y?=w1439:bool)
        n1028 = Negate(x=w1441) -> (-x=w1443:i16)
        n1029 = Select(t=w1443, s="+ phase (APD 2 Gate)", f=w1441) -> (s? t:f=w1440:i16)
        n1030 = Negate(x="Phase Adj. (APD 3 Gate)") -> (-x=w1438:i16)
        n1031 = Or(x="- phase (APD 3 Gate)", y="+ phase (APD 3 Gate)") -> (x .or. y?=w1434:bool)
        n1032 = Select(t=w1438, s="+ phase (APD 3 Gate)", f="Phase Adj. (APD 3 Gate)") -> (s? t:f=w1435:i16)
        n1033 = local read "Phase Adj. (APD Acq)"() -> (w1432:i16)
        n1034 = Or(x="- phase (APD Acq)", y="+ phase (APD Acq)") -> (x .or. y?=w1430:bool)
        n1035 = Negate(x=w1432) -> (-x=w1433:i16)
        n1036 = Select(t=w1433, s="+ phase (APD Acq)", f=w1432) -> (s? t:f=w1431:i16)
        n1037 = xnode "Read/Write Control"("FPGA VI Reference In"=w1453, "error in"=w1452, "Phase count adjustment (APD 1 Gate)"=w1450, "Phase count adjustment (APD 2 Gate)"=w1440, "Phase count adjustment (APD 3 Gate)"=w1435, "Phase Count Adjustment (APD Acq)"=w1431) -> ("FPGA VI Reference Out"=w1448:T20, "error out"=w1449:errorcluster)
        n1038 = xnode "Read/Write Control"("FPGA VI Reference In"=w1448, "error in"=w1449, "+ phase (APD 1 Gate)"=w1446, "+ phase (APD 2 Gate)"=w1439, "+ phase (APD 3 Gate)"=w1434, "+ phase (APD Acq)"=w1430) -> ("error out"=w1447:errorcluster)  [unwired: 1 out]
      }
      event "Invert APD Gate", "APD Gate ON Count", "APD Gate OFF Count", "APD Gate", "APD Integration Time (s)", "APD AO Scale Factor", "Duty Frequency (ON 1/N cycles)", "Interlace ON count", "Interlace OFF count": Value Change {
        n1039 = event-data() -> ()  [unwired: 7 out]
        n1040 = Add(x="Interlace ON count", y="Interlace OFF count") -> (x+y=w1459:u16)
        n1041 = Add(x="APD Gate ON Count", y="APD Gate OFF Count") -> (x+y=w1470:u16)
        n1042 = Multiply(x="Duty Frequency (ON 1/N cycles)", y=w1459) -> (x*y=w1455:u16)
        "Green AI Count" <- w1455
        "Red AI Count" <- w1455
        "Blue AI Count" <- w1455
        n1043 = Subtract(x=w1455, y="Interlace ON count") -> (x-y=w1458:u16)
        n1044 = Multiply(x=w1470, y="Duty Frequency (ON 1/N cycles)") -> (x*y=w1469:u16)
        n1045 = Subtract(x=w1469, y="APD Gate ON Count") -> (x-y=w1468:u16)
        n1046 = local read "DMA Update Period (s)"() -> (w1471:dbl)
        n1047 = Multiply(x="APD Integration Time (s)", y=40000000.0) -> (x*y=w1475:dbl)
        n1048 = Reciprocal(x="APD Integration Time (s)") -> (1/x=→"APD Acq Rate (Hz)":dbl)
        n1049 = To Unsigned Long Integer(number=w1475) -> (unsigned 32bit integer=w1461:u32)
        "APD Int. Count" <- w1461
        n1050 = local read "Number of APDs"() -> (w1454:u8)
        n1051 = Divide(x=w1471, y="APD Integration Time (s)") -> (x/y=w1473:dbl)
        n1052 = Multiply(x=w1454, y=w1473) -> (x*y=w1472:dbl)
        n1053 = local write "APD Samples/FIFO Acq."(w1473) -> ()
        n1054 = local write "APD Elements/DMA read"(w1472) -> ()
        n1055 = xnode "Read/Write Control"("FPGA VI Reference In"=w1479, "error in"=w1478, "Invert APD Gate"="Invert APD Gate", "APD Gate ON Count"="APD Gate ON Count", "APD Gate OFF Count"=w1468, "APD Acq Rate Count"=w1461, "APD Gate Operating Mode"="APD Gate", "APD AO scale factor"="APD AO Scale Factor", "Green interlace ON count"="Interlace ON count", "Green interlace OFF count"=w1458, "Green interlace ON count 2"="Interlace ON count", "Green interlace OFF count 2"=w1458, "Green FB Count"=w1455, "Red interlace ON count"="Interlace ON count", "Red interlace OFF count"="Interlace OFF count", "Blue ON count (AO)"="Interlace ON count", "Blue OFF count (AO)"="Interlace OFF count", "Blue interlace OFF count (D)"="Interlace OFF count", "Blue interlace ON count (D)"="Interlace ON count") -> ("error out"=w1477:errorcluster)  [unwired: 1 out]
      }
      event "Neg. TTrig FPGA": Value Change {
        n1056 = event-data() -> ()  [unwired: 7 out]
        n1057 = xnode "Read/Write Control"("FPGA VI Reference In"=w1482, "error in"=w1481, "TTrig Negate Pos"="Neg. TTrig FPGA") -> ()  [unwired: 2 out]
      }
      event "Test ttrig": Value Change {
        n1058 = event-data() -> ()  [unwired: 7 out]
        n1059 = xnode "Read/Write Control"("FPGA VI Reference In"=w1486, "error in"=w1485, "TTrig?"=TRUE) -> ("error out"=w1484:errorcluster)  [unwired: 1 out]
      }
      event "Number of F/B Scans (AOD)", "Scan Speed (nm/s)", "Scan BD", "Initial delta (MHz)", "Step Size (nm)", "Scan Range (nm)": Value Change {
        w1549 = 123.0  # AOM cal (nm/MHz)
        n1060 = event-data() -> ()  [unwired: 7 out]
        n1061 = local read "BD 1 Frequency 1 (MHz)"() -> (w1532:dbl)
        n1062 = local read "AOM X Cal (nm/MHz)"() -> (w1524:dbl)
        n1063 = local read "X RF Frequency Limits (MHz)"() -> (w1536:T16)
        n1064 = local read "Y RF Frequency Limits (MHz)"() -> (w1533:T16)
        n1065 = local read "BD 2 Frequency 1 (MHz)"() -> (w1538:dbl)
        n1066 = Negate(x="Scan Range (nm)") -> (-x=w1502:dbl)
        n1067 = Divide(x=w1502, y=w1524) -> (x/y=w1506:dbl)
        n1068 = Select(t=w1536, s="Scan BD", f=w1533) -> (s? t:f=w1535:T16)
        n1069 = Select(t=w1532, s="Scan BD", f=w1538) -> (s? t:f=w1537:dbl)
        n1070 = Unbundle By Name(w1535) -> ("Maximum"=w1544:dbl, "Minimum"=w1543:dbl)
        n1071 = Add(x=w1506, y=w1537) -> (x+y=w1541:dbl)
        n1072 = Divide(x=w1502, y="Step Size (nm)") -> (x/y=w1521:dbl)
        n1073 = Divide(x="Step Size (nm)", y=w1524) -> (x/y=w1530:dbl)
        n1074 = Absolute Value(x=w1521) -> (abs(x)=w1505:dbl)
        n1075 = Sign(1:w1502) -> (0:w1503:dbl)
        n1076 = In Range and Coerce(upper limit=w1544, x=w1541, lower limit=w1543) -> (coerced(x)=w1540:dbl, In Range?=w1542:bool)
        n1077 = To Unsigned Quad Integer(1:w1505) -> (0:w1520:u64)
        "Scan steps (AOD)" <- w1520
        n1078 = call "IR AOM freq to word.vi"("Frequency In (MHz)"=w1530) -> ("Frequency Word Out (double)"=w1527:dbl)
        n1079 = Multiply(x=w1503, y=w1527) -> (x*y=w1504:dbl)
        n1080 = Subtract(x=w1541, y=w1540) -> (x-y=w1539:dbl)
        n1081 = To Quad Integer(1:w1504) -> (0:w1526:i64)
        "Incr. int (AOD)" <- w1526
        n1082 = Subtract(x=w1506, y=w1539) -> (x-y=w1525:dbl)
        "Scan Range (MHz)" <- w1525
        n1083 = Select(t=w1506, s=w1542, f=w1525) -> (s? t:f=w1545:dbl)
        n1084 = Multiply(x=w1525, y=w1524) -> (x*y=w1523:dbl)
        n1085 = Decrement(x=w1520) -> (x-1=w1573:u64)
        n1086 = Negate(x=w1523) -> (-x=w1519:dbl)
        n1087 = local write "Scan Range (nm)"(w1519) -> ()
        n1088 = Divide(x=w1545, y=w1573) -> (x/y=w1529:dbl)
        "Scan Increment (MHz)" <- w1529
        n1089 = call "IR AOM freq to word.vi"("Frequency In (MHz)"=w1529) -> ("Frequency Word Out (double)"=w1528:dbl)
        n1090 = Divide(x="Step Size (nm)", y="Scan Speed (nm/s)") -> (x/y=w1516:dbl)
        n1091 = To Quad Integer(1:w1528) -> ()  [unwired: 1 out]
        n1092 = local read "Number Interlace Sets"() -> (w1500:u8)
        n1093 = local read "AI Count (ticks)"() -> (w1501:u16)
        n1094 = local read "Total Counts (ticks)"() -> (w1499:u16)
        n1095 = local read "# Samples/trap"() -> (w1531:u32)
        n1096 = Multiply(x=w1501, y=w1500) -> (x*y=w1498:u16)
        n1097 = Divide(x=w1499, y=w1498) -> (x/y=w1497:dbl)
        n1098 = Select(t=w1532, s="Scan BD", f=w1538) -> (s? t:f=w1570:dbl)
        "Initial freq. (MHz)" <- w1570
        n1099 = Add(x=w1545, y=w1570) -> (x+y=→"Final freq. (MHz)":dbl)
        n1100 = Divide(x=w1499, y=40000000.0) -> (x/y=w1515:dbl)
        n1101 = Divide(x=w1516, y=w1515) -> (x/y=w1514:dbl)
        n1102 = To Unsigned Quad Integer(1:w1514) -> (0:w1489:u64)
        n1103 = Quotient & Remainder(x=w1489, y=u64 2) -> (x-y*floor(x/y)=w1493:u64)  [unwired: 1 out]
        n1104 = Equal?(x=w1493, y=u64 0) -> (x = y?=w1491:bool)
        n1105 = Decrement(x=w1489) -> (x-1=w1490:u64)
        n1106 = Select(t=w1489, s=w1491, f=w1490) -> (s? t:f=w1488:u64)
        "Cycles/step (AOD)" <- w1488
        n1107 = xnode "Read/Write Control"("FPGA VI Reference In"=w1581, "error in"=w1580, "Scan steps"=w1520, "Number of scans"="Number of F/B Scans (AOD)", "Cycles per step"=w1488, "Scan freq.  increment"=w1526, "Scan BD"="Scan BD") -> ("error out"=w1579:errorcluster)  [unwired: 1 out]
        n1108 = Multiply(x=w1520, y=w1488) -> (x*y=w1574:u64)
        n1109 = Multiply(x=w1574, y=u64 2) -> (x*y=w1496:u64)
        n1110 = Multiply(x=w1497, y=w1496) -> (x*y=w1495:dbl)
        "Data points/scan (f/b)" <- w1495
        n1111 = Multiply(x=w1495, y="Number of F/B Scans (AOD)") -> (x*y=w1577:dbl)
        "Data points/scans" <- w1577
        n1112 = Divide(x=w1577, y=w1531) -> (x/y=→"N sets should be saved":dbl)
        n1113 = Multiply(x=w1574, y=w1515) -> (x*y=w1513:dbl)
        "Time/Scan (s) (AOD)" <- w1513
        n1114 = Select(t=w1545, s="Scan BD", f=0.0) -> (s? t:f=w1571:dbl)
        n1115 = Select(t=0.0, s="Scan BD", f=w1545) -> (s? t:f=w1567:dbl)
        n1116 = local read "BD 2 Frequency 2 (MHz)"() -> (w1563:dbl)
        n1117 = local read "BD 1 Frequency 2 (MHz)"() -> (w1566:dbl)
        n1118 = Add(x=w1567, y=w1538) -> (x+y=w1564:dbl)
        n1119 = Add(x=w1532, y=w1571) -> (x+y=w1565:dbl)
        n1120 = Multiply(x=w1513, y=2.0) -> (x*y=w1512:dbl)
        n1121 = Multiply(x=w1512, y="Number of F/B Scans (AOD)") -> (x*y=w1509:dbl)
        n1122 = Divide(x=w1509, y=60.0) -> (x/y=→"Time to Finish All (min)":dbl)
        n1123 = Add(x="Trap 2 Bead Size (nm)", y="Trap 1 Bead Size (nm)") -> (x+y=w1553:dbl)
        n1124 = Divide(x=w1553, y=2.0) -> (x/y=w1547:dbl)
        n1125 = local read "Initial delta (MHz)"() -> (w1550:dbl)
        n1126 = Subtract(x=w1564, y=w1563) -> (x-y=w1561:dbl)
        n1127 = Subtract(x=w1565, y=w1566) -> (x-y=w1562:dbl)
        n1128 = Square(x=w1561) -> (x^2=w1560:dbl)
        n1129 = Square(x=w1562) -> (x^2=w1559:dbl)
        n1130 = Add(x=w1559, y=w1560) -> (x+y=w1558:dbl)
        n1131 = Square Root(x=w1558) -> (sqrt(x)=w1557:dbl)
        "Final delta (MHz)" <- w1557
        n1132 = Multiply(x=w1549, y=w1557) -> (x*y=w1556:dbl)
        n1133 = Multiply(x=w1550, y=w1549) -> (x*y=w1548:dbl)
        n1134 = Subtract(x=w1548, y=w1547) -> (x-y=→"Initial sep (nm)":dbl)
        n1135 = Subtract(x=w1556, y=w1547) -> (x-y=→"Final sep (nm)":dbl)
      }
      event "Freq or Amp switch first", "Swap F1 and F2", "Freq switch delay", "Amp switch delay": Value Change {
        n1136 = event-data() -> ()  [unwired: 7 out]
        n1137 = local read "Amp switch delay"() -> (w1582:u16)
        n1138 = local read "Swap F1 and F2"() -> (w1583:bool)
        n1139 = xnode "Read/Write Control"("FPGA VI Reference In"=w1586, "error in"=w1585, "Swap F1 and F2"=w1583, "Amp switch delay"=w1582) -> ("error out"=w1584:errorcluster)  [unwired: 1 out]
      }
      event "Scan steps (MCL)", "Number of scans (MCL)", "Scan Range (V)\n(of steps)", "2D or 1D Scan", "N APD Samp/step", "Fast Scan Dir", "Continuous MCL Scanning", "Scan lines (y)": Value Change {
        w1588 = 32767.0 ("y")
        n1140 = event-data() -> ()  [unwired: 7 out]
        n1141 = Select(t="Scan lines (y)", s="2D or 1D Scan", f="Number of scans (MCL)") -> (s? t:f=w1593:u64)
        n1142 = Decrement(x="Scan steps (MCL)") -> (x-1=w1609:u64)
        n1143 = Divide(x="Scan Range (V)\n(of steps)", y=w1609) -> (x/y=w1608:dbl)
        "Desired Scan Incr (V)" <- w1608
        n1144 = local read "APD Integration Time (s)"() -> (w1601:dbl)
        n1145 = Multiply(x=w1608, y=w1588) -> (x*y=w1617:dbl)
        n1146 = Divide(x=w1617, y=10.0) -> (x/y=w1607:dbl)
        "Desired incr (int)" <- w1607
        n1147 = local read "Update Count (MCL)"() -> (w1613:u32)
        n1148 = Round Toward -Infinity(1:w1607) -> (0:w1616:dbl)
        n1149 = To Word Integer(number=w1616) -> (16bit integer=w1591:i16)
        "Actual Incr. int (MCL)" <- w1591
        n1150 = Multiply(x=w1601, y=40000000.0) -> (x*y=w1614:dbl)
        n1151 = Divide(x=w1614, y=w1613) -> (x/y=w1612:dbl)
        n1152 = Multiply(x=i16 10, y=w1591) -> (x*y=w1589:i16)
        n1153 = Multiply(x="N APD Samp/step", y=w1612) -> (x*y=w1611:dbl)
        "Cycles/step (MCL)" <- w1611
        n1154 = Divide(x=w1589, y=w1588) -> (x/y=→"Actual MCL Inc (V)":dbl)
        n1155 = Multiply(x="N APD Samp/step", y="Scan steps (MCL)") -> (x*y=w1603:dbl)
        n1156 = local read "APD Samples/FIFO Acq."() -> (w1600:dbl)
        n1157 = Multiply(x=w1603, y=u64 2) -> (x*y=w1602:dbl)
        "Data points/scan (f+b)" <- w1602
        n1158 = Multiply(x=w1602, y=w1593) -> (x*y=w1620:dbl)
        "Data points/scans (MCL)" <- w1620
        n1159 = Multiply(x=w1601, y=w1602) -> (x*y=w1594:dbl)
        "Time/f+b scan (s) (MCL)" <- w1594
        n1160 = Divide(x=w1620, y=w1600) -> (x/y=→"N sets should be saved (MCL)":dbl)
        n1161 = Multiply(x=w1594, y=w1593) -> (x*y=→"Total Time (s)":dbl)
        n1162 = Not(x="Fast Scan Dir") -> (.not. x?=w1598:bool)
        n1163 = xnode "Read/Write Control"("FPGA VI Reference In"=w1624, "error in"=w1623, "Scan steps (MCL)"="Scan steps (MCL)", "Number of scans (MCL)"=w1593, "Cycles per step (MCL)"=w1611, "Scan freq.  increment (MCL)"=w1591, "1D or 2D Scan?"="2D or 1D Scan", "MCL Scan Axis"=w1598, "Cont. Scan (MCL)"="Continuous MCL Scanning") -> ("error out"=w1622:errorcluster)  [unwired: 1 out]
      }
      event "Read Cal": Value Change {
        w1626 = 1000.0 ("y")
        n1164 = event-data() -> ()  [unwired: 7 out]
        n1165 = local read "Save file name"() -> (w1651:path)
        n1166 = local write "Read Cal"(FALSE ("Read Cal")) -> ()
        n1167 = Strip Path(path=w1651) -> (stripped path=w1650:path)  [unwired: 1 out]
        n1168 = Path To String(path=w1650) -> (string=w1649:string)
        n1169 = Concatenate Strings(w1649, "\\current.cal" ("string")) -> (w1647:string)
        n1170 = String To Path(string=w1647) -> (path=w1646:path)
        n1171 = Open/Create/Replace File(file path (use dialog)=w1646, operation (0:open)=T27."open", access (0:read/write)=enum16{"read/write", "read-only", "write-only"}."read-only") -> (refnum out=w1654:refnum<file>, error out=w1640:errorcluster)  [unwired: 1 in, 3 out]
        n1172 = Deny Access(4:w1640, 7:w1654) -> (0:w1639:errorcluster, 3:w1645:refnum<file>)  [unwired: 1 out]
        n1173 = Read from Binary File(5:0.0, 8:w1639, 9:T26."big-endian, network order" ("byte order (0:big-endian, network order)"), 10:-1 ("count (1)"), 11:w1645) -> (0:w1638:errorcluster, 2:w1636:dbl[], 3:w1641:refnum<file>)  [unwired: 2 out]
        n1174 = Array To Cluster(array=w1636) -> (cluster=w1635:T29)
        n1175 = Unbundle(w1635) -> ("[0]"=w1634:dbl, "[1]"=w1633:dbl, "[2]"=w1632:dbl, "[3]"=w1631:dbl, "[4]"=w1630:dbl, "[5]"=w1629:dbl)
        n1176 = Close File(refnum=w1641, error in=w1638) -> (error out=→"Read cal error":errorcluster)  [unwired: 1 out]
        n1177 = Multiply(x=w1629, y=w1626) -> (x*y=w1627:dbl)
        n1178 = local write "T2 kappa_x (pN/nm)"(w1631) -> ()
        n1179 = local write "T1 kappa_x (pN/nm)"(w1632) -> ()
        n1180 = local write "T1 alpha_x (nm/V)"(w1634) -> ()
        n1181 = local write "T2 alpha_x (nm/V)"(w1633) -> ()
        n1182 = Multiply(x=w1630, y=w1626) -> (x*y=w1628:dbl)
        n1183 = local write "T1 offset_x (mV)"(w1628) -> ()
        n1184 = local write "T2 offset_x (mV)"(w1627) -> ()
      }
      event "Abort MCL Scan": Value Change {
        n1185 = event-data() -> ()  [unwired: 7 out]
        n1186 = local write "MCL Scanning"(FALSE ("MCL Scanning")) -> ()
        n1187 = xnode "Read/Write Control"("FPGA VI Reference In"=w1659, "error in"=w1658, "Abort scan (MCL)"="Abort MCL Scan") -> ("error out"=w1657:errorcluster)  [unwired: 1 out]
      }
      event "Update Count (MCL)": Value Change {
        n1188 = event-data() -> ()  [unwired: 7 out]
        n1189 = xnode "Read/Write Control"("FPGA VI Reference In"=w1663, "error in"=w1662, "MCL count"="Update Count (MCL)") -> ("error out"=w1661:errorcluster)  [unwired: 1 out]
      }
      event "+ phase (MCL)", "- phase (MCL)": Value Change {
        n1190 = event-data() -> ()  [unwired: 7 out]
        n1191 = Or(x="- phase (MCL)", y="+ phase (MCL)") -> (x .or. y?=w1666:bool)
        n1192 = Negate(x="Phase adjust (MCL)") -> (-x=w1672:i16)
        n1193 = Select(t=w1672, s="+ phase (MCL)", f="Phase adjust (MCL)") -> (s? t:f=w1670:i16)
        n1194 = xnode "Read/Write Control"("FPGA VI Reference In"=w1674, "error in"=w1673, "Phase count adjustment (MCL)"=w1670) -> ("FPGA VI Reference Out"=w1667:T20, "error out"=w1668:errorcluster)
        n1195 = xnode "Read/Write Control"("FPGA VI Reference In"=w1667, "error in"=w1668, "+ phase (MCL)"=w1666) -> ("error out"=w1665:errorcluster)  [unwired: 1 out]